vi "Dresden R2R Sputter 03.02.2018 IY24.vi"() -> ()   [LabVIEW 2009] (continued)
              }
              frame #8 {
                n6166 = Wait (ms)(milliseconds to wait=u32 500) -> ()  [unwired: 1 out]
              }
              frame #9 {
                n6167 = local write "TC1_speed_coefficient_value"(sgl 0.0 ("TC2_speed_coefficient_value")) -> ()
              }
              frame #10 {
                n6168 = Wait (ms)(milliseconds to wait=u32 100) -> ()  [unwired: 1 out]
              }
              frame #11 {
                n6169 = local write "TC1_speed_coefficient_set"(TRUE ("TC2_speed_coefficient_set")) -> ()
              }
              frame #12 {
                n6170 = Wait (ms)(milliseconds to wait=u32 500) -> ()  [unwired: 1 out]
              }
              frame #13 {
                n6171 = local write "TC1_AO1_polarity(pos_to_neg)"(TRUE ("TC2_AO1_polarity(pos_to_neg)")) -> ()
              }
              frame #14 {
                n6172 = Wait (ms)(milliseconds to wait=u32 500) -> ()  [unwired: 1 out]
              }
              frame #15 {
                n6173 = local write "TC2_close_loop_coefficient"(sgl 0.0 ("TC1_close_loop_coefficient")) -> ()
              }
              frame #16 {
                n6174 = Wait (ms)(milliseconds to wait=u32 100) -> ()  [unwired: 1 out]
              }
              frame #17 {
                n6175 = local write "TC2_close_loop_set"(TRUE ("TC1_close_loop_set")) -> ()
              }
              frame #18 {
                n6176 = Wait (ms)(milliseconds to wait=u32 500) -> ()  [unwired: 1 out]
              }
              frame #19 {
                n6177 = local write "TC2_speed_gain_value"(sgl 0.0 ("TC1_speed_gain_value")) -> ()
              }
              frame #20 {
                n6178 = Wait (ms)(milliseconds to wait=u32 100) -> ()  [unwired: 1 out]
              }
              frame #21 {
                n6179 = local write "TC2_speed_gain_set"(TRUE ("TC1_speed_gain_set")) -> ()
              }
              frame #22 {
                n6180 = Wait (ms)(milliseconds to wait=u32 500) -> ()  [unwired: 1 out]
              }
              frame #23 {
                n6181 = local write "TC2_speed_gain_value"(sgl 28.0 ("TC1_speed_gain_value")) -> ()
              }
              frame #24 {
                n6182 = Wait (ms)(milliseconds to wait=u32 100) -> ()  [unwired: 1 out]
              }
              frame #25 {
                n6183 = local write "TC2_speed_gain_set"(TRUE ("TC1_speed_gain_set")) -> ()
              }
              frame #26 {
                n6184 = Wait (ms)(milliseconds to wait=u32 500) -> ()  [unwired: 1 out]
              }
              frame #27 {
                n6185 = local write "TC2_speed_coefficient_value"(sgl 0.0 ("TC1_speed_coefficient_value")) -> ()
              }
              frame #28 {
                n6186 = Wait (ms)(milliseconds to wait=u32 100) -> ()  [unwired: 1 out]
              }
              frame #29 {
                n6187 = local write "TC2_speed_coefficient_set"(TRUE ("TC1_speed_coefficient_set")) -> ()
              }
              frame #30 {
                n6188 = Wait (ms)(milliseconds to wait=u32 500) -> ()  [unwired: 1 out]
              }
              frame #31 {
                n6189 = local write "TC2_speed_coefficient_value"(sgl 10.0 ("TC1_speed_coefficient_value")) -> ()
              }
              frame #32 {
                n6190 = Wait (ms)(milliseconds to wait=u32 100) -> ()  [unwired: 1 out]
              }
              frame #33 {
                n6191 = local write "TC2_speed_coefficient_set"(TRUE ("TC1_speed_coefficient_set")) -> ()
              }
              frame #34 {
                n6192 = Wait (ms)(milliseconds to wait=u32 500) -> ()  [unwired: 1 out]
              }
              frame #35 {
                n6193 = local write "TC2_AO1_polarity(neg_to_pos)"(TRUE ("TC1_AO1_polarity(neg_to_pos)")) -> ()
              }
              frame #36 {
                n6194 = Wait (ms)(milliseconds to wait=u32 100) -> ()  [unwired: 1 out]
              }
              frame #37 {
                n6195 = local write "TC1_AO1_upper_limit_value"(sgl 10.0 ("TC1_AO1_upper_limit_value")) -> ()
              }
              frame #38 {
                n6196 = Wait (ms)(milliseconds to wait=u32 500) -> ()  [unwired: 1 out]
              }
              frame #39 {
                n6197 = local write "TC1_AO1_upper_limit_set"(TRUE ("TC1_AO1_upper_limit_set")) -> ()
              }
              frame #40 {
                n6198 = Wait (ms)(milliseconds to wait=u32 500) -> ()  [unwired: 1 out]
              }
              frame #41 {
                n6199 = local write "TC2_AO1_upper_limit_value"(sgl 10.0 ("TC2_AO1_upper_limit_value")) -> ()
              }
              frame #42 {
                n6200 = Wait (ms)(milliseconds to wait=u32 500) -> ()  [unwired: 1 out]
              }
              frame #43 {
                n6201 = local write "TC2_AO1_upper_limit_set"(TRUE ("TC2_AO1_upper_limit_set")) -> ()
              }
              frame #44 {
                n6202 = Wait (ms)(milliseconds to wait=u32 500) -> ()  [unwired: 1 out]
              }
              frame #45 {
                n6203 = local write "TC2_AO1_bottom_limit_value"(sgl 0.0 ("TC2_AO1_bottom_limit_value")) -> ()
              }
              frame #46 {
                n6204 = Wait (ms)(milliseconds to wait=u32 500) -> ()  [unwired: 1 out]
              }
              frame #47 {
                n6205 = local write "TC2_AO1_bottom_limit_set"(TRUE ("TC2_AO1_bottom_limit_set")) -> ()
              }
              frame #48 {
                n6206 = Wait (ms)(milliseconds to wait=u32 500) -> ()  [unwired: 1 out]
              }
              frame #49 {
                n6207 = local write "TC1_AO1_bottom_limit_value"(sgl 0.0 ("TC1_AO1_bottom_limit_value")) -> ()
              }
              frame #50 {
                n6208 = Wait (ms)(milliseconds to wait=u32 500) -> ()  [unwired: 1 out]
              }
              frame #51 {
                n6209 = local write "TC1_AO1_bottom_limit_set"(TRUE ("TC1_AO1_bottom_limit_set")) -> ()
              }
              frame #52 {
                w9142 = FALSE ("Parameters_set")
                n6210 = local write "Parameters_set"(w9142) -> ()
                n6211 = local write "Parameters_auto_set"(w9142) -> ()
                n6212 = Wait (ms)(milliseconds to wait=u32 100) -> ()  [unwired: 1 out]
              }
            }
          }
          frame #1 {
            n6213 = stacked-sequence {
              frame #0 {
                n6214 = Wait (ms)(milliseconds to wait=u32 10) -> ()  [unwired: 1 out]
              }
              frame #1 {
                n6215 = local write "TC2_close_loop_coefficient"(sgl 100.0 ("TC2_close_loop_coefficient")) -> ()
              }
              frame #2 {
                n6216 = Wait (ms)(milliseconds to wait=u32 100) -> ()  [unwired: 1 out]
              }
              frame #3 {
                n6217 = local write "TC2_close_loop_set"(TRUE ("TC2_close_loop_set")) -> ()
              }
              frame #4 {
                n6218 = Wait (ms)(milliseconds to wait=u32 500) -> ()  [unwired: 1 out]
              }
              frame #5 {
                n6219 = local write "TC2_speed_gain_value"(sgl 0.0 ("TC2_speed_gain_value")) -> ()
              }
              frame #6 {
                n6220 = Wait (ms)(milliseconds to wait=u32 100) -> ()  [unwired: 1 out]
              }
              frame #7 {
                n6221 = local write "TC2_speed_gain_set"(TRUE ("TC2_speed_gain_set")) -> ()
              }
              frame #8 {
                n6222 = Wait (ms)(milliseconds to wait=u32 500) -> ()  [unwired: 1 out]
              }
              frame #9 {
                n6223 = local write "TC2_speed_coefficient_value"(sgl 0.0 ("TC2_speed_coefficient_value")) -> ()
              }
              frame #10 {
                n6224 = Wait (ms)(milliseconds to wait=u32 100) -> ()  [unwired: 1 out]
              }
              frame #11 {
                n6225 = local write "TC2_speed_coefficient_set"(TRUE ("TC2_speed_coefficient_set")) -> ()
              }
              frame #12 {
                n6226 = Wait (ms)(milliseconds to wait=u32 500) -> ()  [unwired: 1 out]
              }
              frame #13 {
                n6227 = local write "TC2_AO1_polarity(pos_to_neg)"(TRUE ("TC2_AO1_polarity(pos_to_neg)")) -> ()
              }
              frame #14 {
                n6228 = Wait (ms)(milliseconds to wait=u32 500) -> ()  [unwired: 1 out]
              }
              frame #15 {
                n6229 = local write "TC1_close_loop_coefficient"(sgl 0.0 ("TC1_close_loop_coefficient")) -> ()
              }
              frame #16 {
                n6230 = Wait (ms)(milliseconds to wait=u32 100) -> ()  [unwired: 1 out]
              }
              frame #17 {
                n6231 = local write "TC1_close_loop_set"(TRUE ("TC1_close_loop_set")) -> ()
              }
              frame #18 {
                n6232 = Wait (ms)(milliseconds to wait=u32 500) -> ()  [unwired: 1 out]
              }
              frame #19 {
                n6233 = local write "TC1_speed_gain_value"(sgl 0.0 ("TC1_speed_gain_value")) -> ()
              }
              frame #20 {
                n6234 = Wait (ms)(milliseconds to wait=u32 100) -> ()  [unwired: 1 out]
              }
              frame #21 {
                n6235 = local write "TC1_speed_gain_set"(TRUE ("TC1_speed_gain_set")) -> ()
              }
              frame #22 {
                n6236 = Wait (ms)(milliseconds to wait=u32 500) -> ()  [unwired: 1 out]
              }
              frame #23 {
                n6237 = local write "TC1_speed_gain_value"(sgl 28.0 ("TC1_speed_gain_value")) -> ()
              }
              frame #24 {
                n6238 = Wait (ms)(milliseconds to wait=u32 100) -> ()  [unwired: 1 out]
              }
              frame #25 {
                n6239 = local write "TC1_speed_gain_set"(TRUE ("TC1_speed_gain_set")) -> ()
              }
              frame #26 {
                n6240 = Wait (ms)(milliseconds to wait=u32 500) -> ()  [unwired: 1 out]
              }
              frame #27 {
                n6241 = local write "TC1_speed_coefficient_value"(sgl 0.0 ("TC1_speed_coefficient_value")) -> ()
              }
              frame #28 {
                n6242 = Wait (ms)(milliseconds to wait=u32 100) -> ()  [unwired: 1 out]
              }
              frame #29 {
                n6243 = local write "TC1_speed_coefficient_set"(TRUE ("TC1_speed_coefficient_set")) -> ()
              }
              frame #30 {
                n6244 = Wait (ms)(milliseconds to wait=u32 500) -> ()  [unwired: 1 out]
              }
              frame #31 {
                n6245 = local write "TC1_speed_coefficient_value"(sgl 10.0 ("TC1_speed_coefficient_value")) -> ()
              }
              frame #32 {
                n6246 = Wait (ms)(milliseconds to wait=u32 100) -> ()  [unwired: 1 out]
              }
              frame #33 {
                n6247 = local write "TC1_speed_coefficient_set"(TRUE ("TC1_speed_coefficient_set")) -> ()
              }
              frame #34 {
                n6248 = Wait (ms)(milliseconds to wait=u32 500) -> ()  [unwired: 1 out]
              }
              frame #35 {
                n6249 = local write "TC1_AO1_polarity(neg_to_pos)"(TRUE ("TC1_AO1_polarity(neg_to_pos)")) -> ()
              }
              frame #36 {
                n6250 = Wait (ms)(milliseconds to wait=u32 100) -> ()  [unwired: 1 out]
              }
              frame #37 {
                n6251 = local write "TC1_AO1_upper_limit_value"(sgl 10.0 ("TC1_AO1_upper_limit_value")) -> ()
              }
              frame #38 {
                n6252 = Wait (ms)(milliseconds to wait=u32 500) -> ()  [unwired: 1 out]
              }
              frame #39 {
                n6253 = local write "TC1_AO1_upper_limit_set"(TRUE ("TC1_AO1_upper_limit_set")) -> ()
              }
              frame #40 {
                n6254 = Wait (ms)(milliseconds to wait=u32 500) -> ()  [unwired: 1 out]
              }
              frame #41 {
                n6255 = local write "TC1_AO1_bottom_limit_value"(sgl 0.0 ("TC1_AO1_bottom_limit_value")) -> ()
              }
              frame #42 {
                n6256 = Wait (ms)(milliseconds to wait=u32 500) -> ()  [unwired: 1 out]
              }
              frame #43 {
                n6257 = local write "TC1_AO1_bottom_limit_set"(TRUE ("TC1_AO1_bottom_limit_set")) -> ()
              }
              frame #44 {
                n6258 = Wait (ms)(milliseconds to wait=u32 500) -> ()  [unwired: 1 out]
              }
              frame #45 {
                n6259 = local write "TC2_AO1_upper_limit_value"(sgl 10.0 ("TC2_AO1_upper_limit_value")) -> ()
              }
              frame #46 {
                n6260 = Wait (ms)(milliseconds to wait=u32 500) -> ()  [unwired: 1 out]
              }
              frame #47 {
                n6261 = local write "TC2_AO1_upper_limit_set"(TRUE ("TC2_AO1_upper_limit_set")) -> ()
              }
              frame #48 {
                n6262 = Wait (ms)(milliseconds to wait=u32 500) -> ()  [unwired: 1 out]
              }
              frame #49 {
                n6263 = local write "TC2_AO1_bottom_limit_value"(sgl 0.0 ("TC2_AO1_bottom_limit_value")) -> ()
              }
              frame #50 {
                n6264 = Wait (ms)(milliseconds to wait=u32 500) -> ()  [unwired: 1 out]
              }
              frame #51 {
                n6265 = local write "TC2_AO1_bottom_limit_set"(TRUE ("TC2_AO1_bottom_limit_set")) -> ()
              }
              frame #52 {
                w9196 = FALSE ("Parameters_set")
                n6266 = Wait (ms)(milliseconds to wait=u32 100) -> ()  [unwired: 1 out]
                n6267 = local write "Parameters_set"(w9196) -> ()
                n6268 = local write "Parameters_auto_set"(w9196) -> ()
              }
            }
          }
        }
      }
    }
  }
  n6269 = call-poly "VISA Configure Serial Port"(0:"Vat_PC_BV", 7:i16? 7 ("data bits (8)"), 9:w825) -> (4:w827, 15:w828)  [unwired: 11 in]
  n6270 = call-poly "VISA Configure Serial Port"(0:"Pfeiffer TP") -> (4:w830, 15:w829)  [unwired: 6 in, 7 out]
  n6271 = VISA Clear(VISA resource name=w827, error in (no error)=w828) -> (VISA resource name out=w824, error out=w823)
  n6272 = call-poly "VISA Configure Serial Port"(0:"DC_power_supply", 1:i32? 2000 ("timeout (10sec)"), 2:u8 13 ("termination char\n(0xA = '\\n' = LF)"), 3:T/1 ("Enable Termination\nChar (T)"), 5:i32? 19200 ("baud rate (9600)"), 9:w834) -> (4:w838, 15:w839)  [unwired: 3 in, 5 out]
  n6273 = VISA Clear(VISA resource name=w838, error in (no error)=w839) -> (VISA resource name out=w833, error out=w832)
  n6274 = call-poly "VISA Configure Serial Port"(0:"RF", 1:i32? 2000 ("timeout (10sec)"), 2:u8 13 ("termination char\n(0xA = '\\n' = LF)"), 3:T/1 ("Enable Termination\nChar (T)"), 5:i32? 19200 ("baud rate (9600)"), 9:w821) -> (4:w816, 15:w815)  [unwired: 3 in, 5 out]
  n6275 = VISA Clear(VISA resource name=w816, error in (no error)=w815) -> (VISA resource name out=w814, error out=w813)
  n6276 = while {
    tunnel: w824 -> [w9270]
    tunnel: w823 -> [w9269]
    tunnel: [w9267] -> w799
    tunnel: [w9268] -> w798
    stop <- i16? 0 stop-if-true
    n6277 = stacked-sequence {
      tunnel: w9270 -> [w9300 _ _ _]
      tunnel: w9269 -> [w9299 _ _ _]
      tunnel: [_ _ _ w10031] -> w9268
      tunnel: [_ _ _ w10030] -> w9267
      frame #0 {
        n6278 = Or(x="Pc_bv1_set_position", y="Pc_bv1_auto_set position") -> (x .or. y?=w9286)
        n6279 = Compound Arithmetic op=OR("Pc_bv1_open", "Pc_bv1_auto_open", "Pc_bv_open_ch1_gui", "Pc_bv1_open 2") -> (w9281)
        n6280 = Compound Arithmetic op=OR("Pc_bv1_close", "Pc_bv_close_ch1_gui", "Pc_bv1_auto_close", "Pc_bv1_close 2") -> (w9277)
        n6281 = Or(x="Pc_bv1_set_pressure", y="Pc_bv1_auto_set_pressure") -> (x .or. y?=w9288)
        n6282 = Or(x="Baratron_set_zero 4", y="Pc_bv1_auto_baratron_set_zero") -> (x .or. y?=w9287)
        n6283 = Build Array(i16? 0, w9281, w9277, w9286, w9288, w9287, "Learn") -> (w9296)
        n6284 = Boolean Array To Number(Boolean array=w9296) -> (number=w9297)
        n6285 = Mantissa & Exponent(0:w9297) -> (2:w9295)  [unwired: 1 out]
        n6286 = case shown="1" w9295 {
          tunnel: w9300 -> [w9304 w9382 w9406 w9443 w9477 w9501 w9525]
          tunnel: w9299 -> [w9303 w9381 w9405 w9442 w9476 w9500 w9524]
          tunnel: [w9301 w9366 w9390 w9414 w9451 w9485 w9509] -> w9275
          tunnel: [w9302 w9365 w9389 w9413 w9450 w9484 w9508] -> w9276
          frame #0 {
            n6287 = stacked-sequence {
              tunnel: w9304 -> [w9322 _ _ _]
              tunnel: w9303 -> [w9321 _ _ _]
              tunnel: [_ _ w9339 _] -> w9302
              tunnel: [_ _ w9338 _] -> w9301
              frame #0 {
                n6288 = Concatenate Strings("#001A:" ("string"), "\n", "\n") -> (w9324)
                n6289 = VISA Write(VISA resource name=w9322, write buffer=w9324, error in (no error)=w9321) -> (VISA resource name out=w9320, error out=w9319)  [unwired: 1 out]
                n6290 = stacked-sequence {
                  tunnel: [w9329] -> w9318
                  tunnel: w9320 -> [w9329]
                  tunnel: [w9328] -> w9317
                  tunnel: w9319 -> [w9328]
                  frame #0 {
                    n6291 = Wait (ms)(milliseconds to wait=i32? 50) -> ()  [unwired: 1 out]
                  }
                }
                n6292 = property class="Instr"(reference=w9318, error in=w9317) -> (reference out=w9314, error out=w9316, "Serial Settings:Number of Bytes at Serial Port"=w9315)
                n6293 = VISA Read(VISA resource name=w9314, byte count=w9315, error in (no error)=w9316) -> (VISA resource name out=w9307, read buffer=w9305, error out=w9306)  [unwired: 1 out]
                "read buffer 3" <- w9305
                n6294 = Match Pattern(string=w9305, regular expression="#001A:") -> (after substring=w9312)  [unwired: 1 in, 3 out]
                n6295 = String Subset(string=w9312, offset (0)=data[5B], length (rest)=i32? 3 ("length (rest)")) -> (substring=w9309)
                n6296 = Decimal String To Number(string=w9309) -> (number=→"Pc_bv1_position")  [unwired: 2 in, 1 out]
              }
              frame #1 {
                n6297 = Wait (ms)(milliseconds to wait=i32? 10) -> ()  [unwired: 1 out]
              }
              frame #2 {
                n6298 = Concatenate Strings("#001P:" ("string"), "\n", "\n") -> (w9357)
                n6299 = VISA Write(VISA resource name=w9341, write buffer=w9357, error in (no error)=w9340) -> (VISA resource name out=w9356, error out=w9355)  [unwired: 1 out]
                n6300 = stacked-sequence {
                  tunnel: [w9363] -> w9354
                  tunnel: w9356 -> [w9363]
                  tunnel: [w9362] -> w9353
                  tunnel: w9355 -> [w9362]
                  frame #0 {
                    n6301 = Wait (ms)(milliseconds to wait=i32? 50) -> ()  [unwired: 1 out]
                  }
                }
                n6302 = property class="Instr"(reference=w9354, error in=w9353) -> (reference out=w9350, error out=w9352, "Serial Settings:Number of Bytes at Serial Port"=w9351)
                n6303 = VISA Read(VISA resource name=w9350, byte count=w9351, error in (no error)=w9352) -> (VISA resource name out=w9338, read buffer=w9343, error out=w9339)  [unwired: 1 out]
                "read buffer 4" <- w9343
                n6304 = Match Pattern(string=w9343, regular expression="#001P:") -> (after substring=w9334)  [unwired: 1 in, 3 out]
                n6305 = String Subset(string=w9334, offset (0)=data[5B], length (rest)=i32? 1 ("length (rest)")) -> (substring=w9333)
                n6306 = String Subset(string=w9334, offset (0)=i32? 2, length (rest)=i32? 4 ("length (rest)")) -> (substring=w9346)
                n6307 = Equal?(x=w9333, y="-") -> (x = y?=w9331)
                n6308 = Decimal String To Number(string=w9346) -> (number=w9345)  [unwired: 2 in, 1 out]
                n6309 = case shown="True" w9331 {
                  frame #0 {
                  }
                  frame #1 {
                    w9360 = data[9B] ("Pressure")
                    n6310 = local write "Pressure"(w9360) -> ()
                    n6311 = local write "Pressure_gui"(w9360) -> ()
                    n6312 = local write "Pressure_gui 2"(w9360) -> ()
                  }
                }
                n6313 = Divide(x=w9345, y=i32? 100) -> (x/y=→"Pressure" →"Pressure_gui" →"Pressure_gui 2")
              }
              frame #3 {
                n6314 = Wait (ms)(milliseconds to wait=i32? 10) -> ()  [unwired: 1 out]
              }
            }
          }
          frame #1 {
            n6315 = Concatenate Strings("#001O:" ("string"), "\n", "\n") -> (w9378)
            n6316 = VISA Write(VISA resource name=w9382, write buffer=w9378, error in (no error)=w9381) -> (VISA resource name out=w9370, error out=w9369)  [unwired: 1 out]
            n6317 = local write "Pc_bv1_auto_open"(i16? 0 ("Pc_bv1_auto_open")) -> ()
            n6318 = stacked-sequence {
              tunnel: [w9388] -> w9375
              tunnel: w9370 -> [w9388]
              tunnel: [w9387] -> w9374
              tunnel: w9369 -> [w9387]
              frame #0 {
                n6319 = Wait (ms)(milliseconds to wait=i32? 50) -> ()  [unwired: 1 out]
              }
            }
            n6320 = property class="Instr"(reference=w9375, error in=w9374) -> (reference out=w9371, error out=w9373, "Serial Settings:Number of Bytes at Serial Port"=w9372)
            n6321 = VISA Read(VISA resource name=w9371, byte count=w9372, error in (no error)=w9373) -> (VISA resource name out=w9368, error out=w9367)  [unwired: 2 out]
            n6322 = stacked-sequence {
              tunnel: [w9385] -> w9366
              tunnel: w9368 -> [w9385]
              tunnel: [w9384] -> w9365
              tunnel: w9367 -> [w9384]
              frame #0 {
                n6323 = Wait (ms)(milliseconds to wait=i32? 50) -> ()  [unwired: 1 out]
              }
            }
          }
          frame #2 {
            n6324 = Concatenate Strings("#001C:" ("string"), "\n", "\n") -> (w9402)
            n6325 = local write "Pc_bv1_auto_close"(i16? 0 ("Pc_bv1_auto_close")) -> ()
            n6326 = VISA Write(VISA resource name=w9406, write buffer=w9402, error in (no error)=w9405) -> (VISA resource name out=w9391, error out=w9392)  [unwired: 1 out]
            n6327 = stacked-sequence {
              tunnel: [w9412] -> w9399
              tunnel: w9391 -> [w9412]
              tunnel: [w9411] -> w9398
              tunnel: w9392 -> [w9411]
              frame #0 {
                n6328 = Wait (ms)(milliseconds to wait=i32? 50) -> ()  [unwired: 1 out]
              }
            }
            n6329 = property class="Instr"(reference=w9399, error in=w9398) -> (reference out=w9395, error out=w9397, "Serial Settings:Number of Bytes at Serial Port"=w9396)
            n6330 = VISA Read(VISA resource name=w9395, byte count=w9396, error in (no error)=w9397) -> (VISA resource name out=w9394, error out=w9393)  [unwired: 2 out]
            n6331 = stacked-sequence {
              tunnel: [w9409] -> w9390
              tunnel: w9394 -> [w9409]
              tunnel: [w9408] -> w9389
              tunnel: w9393 -> [w9408]
              frame #0 {
                n6332 = Wait (ms)(milliseconds to wait=i32? 50) -> ()  [unwired: 1 out]
              }
            }
          }
          frame #3 {
            n6333 = In Range and Coerce(upper limit=dbl? 100.0, x="Set_position_value", lower limit=data[9B]) -> (coerced(x)=w9433)  [unwired: 1 out]
            n6334 = Multiply(x=w9433, y=dbl? 1000.0) -> (x*y=w9430)
            n6335 = Number To Decimal String(number=w9430) -> (decimal integer string=w9431)  [unwired: 1 out]
            n6336 = Concatenate Strings("000000" ("string"), w9431) -> (w9425)
            n6337 = String Length(string=w9425) -> (length=w9427)
            n6338 = Subtract(x=w9427, y=i32? 6) -> (x-y=w9429)
            n6339 = String Subset(string=w9425, offset (0)=w9429) -> (substring=w9424)  [unwired: 1 out]
            n6340 = Concatenate Strings("#001R:" ("string"), w9424, "\n", "\n") -> (w9441)
            n6341 = VISA Write(VISA resource name=w9443, write buffer=w9441, error in (no error)=w9442) -> (VISA resource name out=w9416, error out=w9415)  [unwired: 1 out]
            n6342 = stacked-sequence {
              tunnel: [w9449] -> w9423
              tunnel: w9416 -> [w9449]
              tunnel: [w9448] -> w9422
              tunnel: w9415 -> [w9448]
              frame #0 {
                n6343 = Wait (ms)(milliseconds to wait=i32? 50) -> ()  [unwired: 1 out]
              }
            }
            n6344 = property class="Instr"(reference=w9423, error in=w9422) -> (reference out=w9419, error out=w9421, "Serial Settings:Number of Bytes at Serial Port"=w9420)
            n6345 = VISA Read(VISA resource name=w9419, byte count=w9420, error in (no error)=w9421) -> (VISA resource name out=w9418, error out=w9417)  [unwired: 2 out]
            n6346 = local write "Pc_bv1_auto_set position"(i16? 0 ("Pc_bv1_auto_set position")) -> ()
            n6347 = stacked-sequence {
              tunnel: [w9446] -> w9414
              tunnel: w9418 -> [w9446]
              tunnel: [w9445] -> w9413
              tunnel: w9417 -> [w9445]
              frame #0 {
                n6348 = Wait (ms)(milliseconds to wait=i32? 50) -> ()  [unwired: 1 out]
              }
            }
          }
          frame #4 {
            n6349 = Multiply(x="Set_pressure_value", y=dbl? 10000.0) -> (x*y=w9468)
            n6350 = Number To Decimal String(number=w9468) -> (decimal integer string=w9462)  [unwired: 1 out]
            n6351 = Concatenate Strings("00000000" ("string"), w9462) -> (w9464)
            n6352 = String Length(string=w9464) -> (length=w9465)
            n6353 = Subtract(x=w9465, y=i32? 8) -> (x-y=w9467)
            n6354 = String Subset(string=w9464, offset (0)=w9467) -> (substring=w9461)  [unwired: 1 out]
            n6355 = Concatenate Strings("#001S:" ("string"), w9461, "\n", "\n") -> (w9469)
            n6356 = VISA Write(VISA resource name=w9477, write buffer=w9469, error in (no error)=w9476) -> (VISA resource name out=w9453, error out=w9452)  [unwired: 1 out]
            n6357 = stacked-sequence {
              tunnel: [w9483] -> w9460
              tunnel: w9453 -> [w9483]
              tunnel: [w9482] -> w9459
              tunnel: w9452 -> [w9482]
              frame #0 {
                n6358 = Wait (ms)(milliseconds to wait=i32? 50) -> ()  [unwired: 1 out]
              }
            }
            n6359 = property class="Instr"(reference=w9460, error in=w9459) -> (reference out=w9456, error out=w9458, "Serial Settings:Number of Bytes at Serial Port"=w9457)
            n6360 = VISA Read(VISA resource name=w9456, byte count=w9457, error in (no error)=w9458) -> (VISA resource name out=w9455, error out=w9454)  [unwired: 2 out]
            n6361 = stacked-sequence {
              tunnel: [w9480] -> w9451
              tunnel: w9455 -> [w9480]
              tunnel: [w9479] -> w9450
              tunnel: w9454 -> [w9479]
              frame #0 {
                n6362 = Wait (ms)(milliseconds to wait=i32? 50) -> ()  [unwired: 1 out]
              }
            }
            n6363 = local write "Pc_bv1_auto_set_pressure"(i16? 0 ("Pc_bv1_auto_set_pressure")) -> ()
          }
          frame #5 {
            n6364 = local write "Pc_bv1_auto_baratron_set_zero"(i16? 0 ("Pc_bv1_auto_baratron_set_zero")) -> ()
            n6365 = Concatenate Strings("#001Z:" ("string"), "\n", "\n") -> (w9497)
            n6366 = VISA Write(VISA resource name=w9501, write buffer=w9497, error in (no error)=w9500) -> (VISA resource name out=w9487, error out=w9486)  [unwired: 1 out]
            n6367 = stacked-sequence {
              tunnel: [w9507] -> w9494
              tunnel: w9487 -> [w9507]
              tunnel: [w9506] -> w9493
              tunnel: w9486 -> [w9506]
              frame #0 {
                n6368 = Wait (ms)(milliseconds to wait=i32? 50) -> ()  [unwired: 1 out]
              }
            }
            n6369 = property class="Instr"(reference=w9494, error in=w9493) -> (reference out=w9490, error out=w9492, "Serial Settings:Number of Bytes at Serial Port"=w9491)
            n6370 = VISA Read(VISA resource name=w9490, byte count=w9491, error in (no error)=w9492) -> (VISA resource name out=w9489, error out=w9488)  [unwired: 2 out]
            n6371 = stacked-sequence {
              tunnel: [w9504] -> w9485
              tunnel: w9489 -> [w9504]
              tunnel: [w9503] -> w9484
              tunnel: w9488 -> [w9503]
              frame #0 {
                n6372 = Wait (ms)(milliseconds to wait=i32? 50) -> ()  [unwired: 1 out]
              }
            }
          }
          frame #6 {
            n6373 = Concatenate Strings("#001L:" ("string"), "Learn value", "\n", "\n") -> (w9521)
            n6374 = VISA Write(VISA resource name=w9525, write buffer=w9521, error in (no error)=w9524) -> (VISA resource name out=w9511, error out=w9510)  [unwired: 1 out]
            n6375 = stacked-sequence {
              tunnel: [w9531] -> w9518
              tunnel: w9511 -> [w9531]
              tunnel: [w9530] -> w9517
              tunnel: w9510 -> [w9530]
              frame #0 {
                n6376 = Wait (ms)(milliseconds to wait=i32? 50) -> ()  [unwired: 1 out]
              }
            }
            n6377 = property class="Instr"(reference=w9518, error in=w9517) -> (reference out=w9514, error out=w9516, "Serial Settings:Number of Bytes at Serial Port"=w9515)
            n6378 = VISA Read(VISA resource name=w9514, byte count=w9515, error in (no error)=w9516) -> (VISA resource name out=w9513, error out=w9512)  [unwired: 2 out]
            n6379 = stacked-sequence {
              tunnel: [w9528] -> w9509
              tunnel: w9513 -> [w9528]
              tunnel: [w9527] -> w9508
              tunnel: w9512 -> [w9527]
              frame #0 {
                n6380 = Wait (ms)(milliseconds to wait=i32? 50) -> ()  [unwired: 1 out]
              }
            }
          }
        }
      }
      frame #1 {
        n6381 = Or(x="Pc_bv2_set_position", y="Pc_bv2_auto_set position") -> (x .or. y?=w9554)
        n6382 = Or(x="Pc_bv2_set_pressure", y="Pc_bv2_auto_set_pressure") -> (x .or. y?=w9553)
        n6383 = Compound Arithmetic op=OR("Pc_bv2_open 2", "Pc_bv2_open", "Pc_bv_open_ch2_gui", "Pc_bv2_auto_open") -> (w9539)
        n6384 = Compound Arithmetic op=OR("Pc_bv2_close 2", "Pc_bv2_close", "Pc_bv2_auto_close", "Pc_bv_close_ch2_gui") -> (w9538)
        n6385 = Or(x="Baratron_set_zero 2", y="Pc_bv2_auto_baratron_set_zero") -> (x .or. y?=w9552)
        n6386 = Build Array(i16? 0, w9539, w9538, w9554, w9553, w9552) -> (w9556)
        n6387 = Boolean Array To Number(Boolean array=w9556) -> (number=w9558)
        n6388 = Mantissa & Exponent(0:w9558) -> (2:w9557)  [unwired: 1 out]
        n6389 = case shown="4" w9557 {
          tunnel: [w9562 w9626 w9649 w9672 w9709 w9744] -> w9536
          tunnel: [w9561 w9627 w9648 w9673 w9710 w9743] -> w9535
          tunnel: w9537 -> [w9560 w9636 w9660 w9684 w9721 w9755]
          tunnel: w9534 -> [w9559 w9635 w9659 w9683 w9720 w9754]
          frame #0 {
            n6390 = stacked-sequence {
              tunnel: [_ _ _ w9602 _] -> w9562
              tunnel: [_ _ _ w9601 _] -> w9561
              tunnel: w9560 -> [_ w9565 _ _ _]
              tunnel: w9559 -> [_ w9564 _ _ _]
              frame #0 {
                n6391 = Wait (ms)(milliseconds to wait=i32? 50) -> ()  [unwired: 1 out]
              }
              frame #1 {
                n6392 = Concatenate Strings("#002A:" ("string"), "\n", "\n") -> (w9583)
                n6393 = VISA Write(VISA resource name=w9565, write buffer=w9583, error in (no error)=w9564) -> (VISA resource name out=w9581, error out=w9580)  [unwired: 1 out]
                n6394 = stacked-sequence {
                  tunnel: [w9588] -> w9579
                  tunnel: w9581 -> [w9588]
                  tunnel: [w9587] -> w9578
                  tunnel: w9580 -> [w9587]
                  frame #0 {
                    n6395 = Wait (ms)(milliseconds to wait=i32? 50) -> ()  [unwired: 1 out]
                  }
                }
                n6396 = property class="Instr"(reference=w9579, error in=w9578) -> (reference out=w9575, error out=w9577, "Serial Settings:Number of Bytes at Serial Port"=w9576)
                n6397 = VISA Read(VISA resource name=w9575, byte count=w9576, error in (no error)=w9577) -> (VISA resource name out=w9567, read buffer=w9569, error out=w9566)  [unwired: 1 out]
                "read buffer 2" <- w9569
                n6398 = Match Pattern(string=w9569, regular expression="#002A:") -> (after substring=w9573)  [unwired: 1 in, 3 out]
                n6399 = String Subset(string=w9573, offset (0)=data[5B], length (rest)=i32? 3 ("length (rest)")) -> (substring=w9570)
                n6400 = Decimal String To Number(string=w9570) -> (number=→"Pc_bv2_position")  [unwired: 2 in, 1 out]
              }
              frame #2 {
                n6401 = Wait (ms)(milliseconds to wait=i32? 50) -> ()  [unwired: 1 out]
              }
              frame #3 {
                n6402 = Concatenate Strings("#002P:" ("string"), "\n", "\n") -> (w9616)
                n6403 = VISA Write(VISA resource name=w9600, write buffer=w9616, error in (no error)=w9599) -> (VISA resource name out=w9614, error out=w9613)  [unwired: 1 out]
                n6404 = stacked-sequence {
                  tunnel: [w9622] -> w9612
                  tunnel: w9614 -> [w9622]
                  tunnel: [w9621] -> w9611
                  tunnel: w9613 -> [w9621]
                  frame #0 {
                    n6405 = Wait (ms)(milliseconds to wait=i32? 50) -> ()  [unwired: 1 out]
                  }
                }
                n6406 = property class="Instr"(reference=w9612, error in=w9611) -> (reference out=w9608, error out=w9610, "Serial Settings:Number of Bytes at Serial Port"=w9609)
                n6407 = VISA Read(VISA resource name=w9608, byte count=w9609, error in (no error)=w9610) -> (VISA resource name out=w9602, read buffer=w9603, error out=w9601)  [unwired: 1 out]
                "read buffer 5" <- w9603
                n6408 = Match Pattern(string=w9603, regular expression="#002P:") -> (after substring=w9590)  [unwired: 1 in, 3 out]
                n6409 = String Subset(string=w9590, offset (0)=data[5B], length (rest)=i32? 1 ("length (rest)")) -> (substring=w9593)
                n6410 = String Subset(string=w9590, offset (0)=i32? 2, length (rest)=i32? 4 ("length (rest)")) -> (substring=w9604)
                n6411 = Equal?(x=w9593, y="-") -> (x = y?=w9591)
                n6412 = Decimal String To Number(string=w9604) -> (number=w9598)  [unwired: 2 in, 1 out]
                n6413 = case shown="True" w9591 {
                  frame #0 {
                  }
                  frame #1 {
                    w9619 = data[5B] ("Pressure 2")
                    n6414 = local write "Pressure 2_gui"(w9619) -> ()
                    n6415 = local write "Pressure 2_gui 2"(w9619) -> ()
                    n6416 = local write "Pressure 2"(w9619) -> ()
                  }
                }
                n6417 = Divide(x=w9598, y=i32? 100) -> (x/y=→"Pressure 2" →"Pressure 2_gui" →"Pressure 2_gui 2")
              }
              frame #4 {
                n6418 = Wait (ms)(milliseconds to wait=i32? 50) -> ()  [unwired: 1 out]
              }
            }
          }
          frame #1 {
            n6419 = Concatenate Strings("#002O:" ("string"), "\n", "\n") -> (w9639)
            n6420 = VISA Write(VISA resource name=w9636, write buffer=w9639, error in (no error)=w9635) -> (VISA resource name out=w9624, error out=w9625)  [unwired: 1 out]
            n6421 = stacked-sequence {
              tunnel: [w9647] -> w9634
              tunnel: w9624 -> [w9647]
              tunnel: [w9646] -> w9633
              tunnel: w9625 -> [w9646]
              frame #0 {
                n6422 = Wait (ms)(milliseconds to wait=i32? 50) -> ()  [unwired: 1 out]
              }
            }
            n6423 = local write "Pc_bv2_auto_open"(i16? 0 ("Pc_bv2_auto_open")) -> ()
            n6424 = property class="Instr"(reference=w9634, error in=w9633) -> (reference out=w9630, error out=w9632, "Serial Settings:Number of Bytes at Serial Port"=w9631)
            n6425 = VISA Read(VISA resource name=w9630, byte count=w9631, error in (no error)=w9632) -> (VISA resource name out=w9629, error out=w9628)  [unwired: 2 out]
            n6426 = stacked-sequence {
              tunnel: [w9644] -> w9626
              tunnel: w9629 -> [w9644]
              tunnel: [w9643] -> w9627
              tunnel: w9628 -> [w9643]
              frame #0 {
                n6427 = Wait (ms)(milliseconds to wait=i32? 50) -> ()  [unwired: 1 out]
              }
            }
          }
          frame #2 {
            n6428 = Concatenate Strings("#002C:" ("string"), "\n", "\n") -> (w9663)
            n6429 = VISA Write(VISA resource name=w9660, write buffer=w9663, error in (no error)=w9659) -> (VISA resource name out=w9651, error out=w9650)  [unwired: 1 out]
            n6430 = local write "Pc_bv2_auto_close"(i16? 0 ("Pc_bv2_auto_close")) -> ()
            n6431 = stacked-sequence {
              tunnel: [w9671] -> w9658
              tunnel: w9651 -> [w9671]
              tunnel: [w9670] -> w9657
              tunnel: w9650 -> [w9670]
              frame #0 {
                n6432 = Wait (ms)(milliseconds to wait=i32? 50) -> ()  [unwired: 1 out]
              }
            }
            n6433 = property class="Instr"(reference=w9658, error in=w9657) -> (reference out=w9654, error out=w9656, "Serial Settings:Number of Bytes at Serial Port"=w9655)
            n6434 = VISA Read(VISA resource name=w9654, byte count=w9655, error in (no error)=w9656) -> (VISA resource name out=w9653, error out=w9652)  [unwired: 2 out]
            n6435 = stacked-sequence {
              tunnel: [w9668] -> w9649
              tunnel: w9653 -> [w9668]
              tunnel: [w9667] -> w9648
              tunnel: w9652 -> [w9667]
              frame #0 {
                n6436 = Wait (ms)(milliseconds to wait=i32? 50) -> ()  [unwired: 1 out]
              }
            }
          }
          frame #3 {
            n6437 = In Range and Coerce(upper limit=dbl? 100.0, x="Set_position_value 2", lower limit=data[9B]) -> (coerced(x)=w9686)  [unwired: 1 out]
            n6438 = Multiply(x=w9686, y=dbl? 1000.0) -> (x*y=w9693)
            n6439 = Number To Decimal String(number=w9693) -> (decimal integer string=w9695)  [unwired: 1 out]
            n6440 = Concatenate Strings("000000" ("string"), w9695) -> (w9697)
            n6441 = String Length(string=w9697) -> (length=w9698)
            n6442 = Subtract(x=w9698, y=i32? 6) -> (x-y=w9700)
            n6443 = String Subset(string=w9697, offset (0)=w9700) -> (substring=w9690)  [unwired: 1 out]
            n6444 = Concatenate Strings("#002R:" ("string"), w9690, "\n", "\n") -> (w9702)
            n6445 = VISA Write(VISA resource name=w9684, write buffer=w9702, error in (no error)=w9683) -> (VISA resource name out=w9676, error out=w9675)  [unwired: 1 out]
            n6446 = stacked-sequence {
              tunnel: [w9707] -> w9677
              tunnel: w9676 -> [w9707]
              tunnel: [w9706] -> w9674
              tunnel: w9675 -> [w9706]
              frame #0 {
                n6447 = Wait (ms)(milliseconds to wait=i32? 50) -> ()  [unwired: 1 out]
              }
            }
            n6448 = property class="Instr"(reference=w9677, error in=w9674) -> (reference out=w9680, error out=w9682, "Serial Settings:Number of Bytes at Serial Port"=w9681)
            n6449 = VISA Read(VISA resource name=w9680, byte count=w9681, error in (no error)=w9682) -> (VISA resource name out=w9679, error out=w9678)  [unwired: 2 out]
            n6450 = local write "Pc_bv2_auto_set position"(i16? 0 ("Pc_bv2_auto_set position")) -> ()
            n6451 = stacked-sequence {
              tunnel: [w9705] -> w9672
              tunnel: w9679 -> [w9705]
              tunnel: [w9704] -> w9673
              tunnel: w9678 -> [w9704]
              frame #0 {
                n6452 = Wait (ms)(milliseconds to wait=i32? 50) -> ()  [unwired: 1 out]
              }
            }
          }
          frame #4 {
            n6453 = Multiply(x="Set_pressure_value 2", y=dbl? 10000.0) -> (x*y=w9727)
            n6454 = Number To Decimal String(number=w9727) -> (decimal integer string=w9729)  [unwired: 1 out]
            n6455 = Concatenate Strings("00000000" ("string"), w9729) -> (w9731)
            n6456 = String Length(string=w9731) -> (length=w9732)
            n6457 = Subtract(x=w9732, y=i32? 8) -> (x-y=w9734)
            n6458 = String Subset(string=w9731, offset (0)=w9734) -> (substring=w9724)  [unwired: 1 out]
            n6459 = Concatenate Strings("#002S:" ("string"), w9724, "\n", "\n") -> (w9736)
            n6460 = VISA Write(VISA resource name=w9721, write buffer=w9736, error in (no error)=w9720) -> (VISA resource name out=w9712, error out=w9711)  [unwired: 1 out]
            n6461 = stacked-sequence {
              tunnel: [w9741] -> w9714
              tunnel: w9712 -> [w9741]
              tunnel: [w9740] -> w9713
              tunnel: w9711 -> [w9740]
              frame #0 {
                n6462 = Wait (ms)(milliseconds to wait=i32? 50) -> ()  [unwired: 1 out]
              }
            }
            n6463 = property class="Instr"(reference=w9714, error in=w9713) -> (reference out=w9717, error out=w9719, "Serial Settings:Number of Bytes at Serial Port"=w9718)
            n6464 = VISA Read(VISA resource name=w9717, byte count=w9718, error in (no error)=w9719) -> (VISA resource name out=w9716, error out=w9715)  [unwired: 2 out]
            n6465 = local write "Pc_bv2_auto_set_pressure"(i16? 0 ("Pc_bv2_auto_set_pressure")) -> ()
            n6466 = stacked-sequence {
              tunnel: [w9739] -> w9709
              tunnel: w9716 -> [w9739]
              tunnel: [w9738] -> w9710
              tunnel: w9715 -> [w9738]
              frame #0 {
                n6467 = Wait (ms)(milliseconds to wait=i32? 50) -> ()  [unwired: 1 out]
              }
            }
          }
          frame #5 {
            n6468 = Concatenate Strings("#002Z:" ("string"), "\n", "\n") -> (w9758)
            n6469 = VISA Write(VISA resource name=w9755, write buffer=w9758, error in (no error)=w9754) -> (VISA resource name out=w9746, error out=w9745)  [unwired: 1 out]
            n6470 = stacked-sequence {
              tunnel: [w9765] -> w9748
              tunnel: w9746 -> [w9765]
              tunnel: [w9764] -> w9747
              tunnel: w9745 -> [w9764]
              frame #0 {
                n6471 = Wait (ms)(milliseconds to wait=i32? 50) -> ()  [unwired: 1 out]
              }
            }
            n6472 = property class="Instr"(reference=w9748, error in=w9747) -> (reference out=w9751, error out=w9753, "Serial Settings:Number of Bytes at Serial Port"=w9752)
            n6473 = local write "Pc_bv2_auto_baratron_set_zero"(i16? 0 ("Pc_bv2_auto_baratron_set_zero")) -> ()
            n6474 = VISA Read(VISA resource name=w9751, byte count=w9752, error in (no error)=w9753) -> (VISA resource name out=w9750, error out=w9749)  [unwired: 2 out]
            n6475 = stacked-sequence {
              tunnel: [w9763] -> w9744
              tunnel: w9750 -> [w9763]
              tunnel: [w9762] -> w9743
              tunnel: w9749 -> [w9762]
              frame #0 {
                n6476 = Wait (ms)(milliseconds to wait=i32? 50) -> ()  [unwired: 1 out]
              }
            }
          }
        }
      }
      frame #2 {
        n6477 = Compound Arithmetic op=OR("Pc_bv3_open 2", "Pc_bv3_open", "Pc_bv_open_ch3_gui", "Pc_bv3_auto_open") -> (w9777)
        n6478 = Or(x="Pc_bv3_set_pressure", y="Pc_bv3_auto_set_pressure") -> (x .or. y?=w9787)
        n6479 = Compound Arithmetic op=OR("Pc_bv3_close 2", "Pc_bv3_close", "Pc_bv_close_ch3_gui", "Pc_bv3_auto_close") -> (w9773)
        n6480 = Or(x="Pc_bv3_set_position", y="Pc_bv3_auto_set position") -> (x .or. y?=w9788)
        n6481 = Or(x="Pc_bv3_auto_baratron_set_zero", y="Baratron_set_zero 3") -> (x .or. y?=w9784)
        n6482 = Build Array(i16? 0, w9777, w9773, w9788, w9787, w9784) -> (w9791)
        n6483 = Boolean Array To Number(Boolean array=w9791) -> (number=w9793)
        n6484 = Mantissa & Exponent(0:w9793) -> (2:w9792)  [unwired: 1 out]
        n6485 = case shown="4" w9792 {
          tunnel: [w9797 w9859 w9884 w9908 w9945 w9979 w10003] -> w9771
          tunnel: [w9796 w9861 w9883 w9907 w9944 w9978 w10002] -> w9770